vi "for testing.vi"() -> ()   [LabVIEW 2016] (continued)
            n234 = call "uc480_Error_Handling.vi"("Error Code"=w445, "Error String"=w454, "Error In"=w443) -> ("Error Out"=w447:errorcluster)  [unwired: 8 in]
          }
          frame True {
          }
        }
        n235 = call "uc480_SubVI_Example_MemoryAllocation.vi"(".NET (Reference)"=w406, "Error In"=w431) -> ("Error Out"=w408:errorcluster)  [unwired: 13 in, 4 out]
        n236 = call "uc480_SubVI_Example_GetPixelClock.vi"(".NET (Reference)"=w406, "Error In"=w408) -> ("Pixel Clock"=w409:i32, "Inc"=w411:i32, "Min"=w412:i32, "Max"=w413:i32, "error out"=w410:errorcluster)  [unwired: 9 in]
        n237 = property on="Pixelclock" class="Slide (strict)"(error in=w410, "Value"=w409, "Increment"=w411, "Minimum"=w412, "Maximum"=w413) -> (error out=w414:errorcluster)  [unwired: 1 in, 1 out]
        n238 = property on="Pixelclock" class="Slide (strict)"(error in=w414, "Scale.Increment"=w411, "Scale.Minimum"=w412, "Scale.Maximum"=w413) -> (error out=w415:errorcluster)  [unwired: 1 in, 1 out]
        n239 = call "uc480_SubVI_Example_GetFramerate.vi"(".NET (Reference)"=w406, "Error In"=w415) -> ("Framerate"=w418:dbl, "Inc"=w419:dbl, "Min"=w420:dbl, "Max"=w421:dbl, "error out"=w417:errorcluster)  [unwired: 9 in]
        n240 = property on="Framerate" class="Slide (strict)"(error in=w417, "Value"=w418, "Increment"=w419, "Minimum"=w420, "Maximum"=w421) -> (error out=w416:errorcluster)  [unwired: 1 in, 1 out]
        n241 = property on="Framerate" class="Slide (strict)"(error in=w416, "Scale.Increment"=w419, "Scale.Minimum"=w420, "Scale.Maximum"=w421) -> (error out=w422:errorcluster)  [unwired: 1 in, 1 out]
        n242 = call "uc480_SubVI_Example_GetExposure.vi"(".NET (Reference)"=w406, "Error In"=w422) -> ("Exposure"=w425:dbl, "Inc"=w426:dbl, "Min"=w427:dbl, "Max"=w428:dbl, "Error out"=w423:errorcluster)  [unwired: 9 in]
        n243 = property on="Exposure" class="Slide (strict)"(error in=w423, "Value"=w425, "Increment"=w426, "Minimum"=w427, "Maximum"=w428) -> (error out=w424:errorcluster)  [unwired: 1 in, 1 out]
        n244 = property on="Exposure" class="Slide (strict)"(error in=w424, "Scale.Increment"=w426, "Scale.Minimum"=w427, "Scale.Maximum"=w428) -> (error out=w407:errorcluster)  [unwired: 1 in, 1 out]
      }
      frame "Stop live" {
        # "Is acquisition running?"
        # "Stop Acquisition"
        n245 = property class="Camera"(reference=w472, error in=w473) -> (error out=w480:errorcluster, "Acquisition"=w479:refnum<k24>)  [unwired: 1 out]
        n246 = invoke class="Acquisition" method="HasStarted"(reference=w479, error in=w480) -> (reference out=w474:refnum<k24>, error out=w476:errorcluster, "bValue"=w478:bool)  [unwired: 2 in, 1 out]
        n247 = control-ref of="Load Parameter"() -> (w468:refnum<vi>)
        n248 = control-ref of="Start Live"() -> (w465:refnum<vi>)
        n249 = invoke class="Acquisition" method="ToString"(reference=w474, error in=w476) -> (reference out=w457:refnum<k24>, error out=w459:errorcluster, "ToString"=w475:string)  [unwired: 1 in]
        n250 = property class="Bool"(reference=w468, "Disabled"=u8 0 ("Deaktiviert")) -> (reference out=w463:refnum<vi>, error out=w462:errorcluster)  [unwired: 1 in]
        n251 = property class="Bool"(reference=w465, "Disabled"=u8 0 ("Deaktiviert")) -> (reference out=w461:refnum<vi>, error out=w460:errorcluster)  [unwired: 1 in]
        n252 = Close Reference(reference=w457, error in (no error)=w459) -> (error out=w458:errorcluster)
        n253 = Close Reference(reference=w463, error in (no error)=w462) -> ()  [unwired: 1 out]
        n254 = Close Reference(reference=w461, error in (no error)=w460) -> ()  [unwired: 1 out]
        n255 = call "uc480_Error_Handling.vi"("Error String"=w475, "Error In"=w458) -> ("Error Out"=w477:errorcluster)  [unwired: 9 in]
        n256 = case shown="True" w478 {
          tunnel: [w482 w501] -> w470
          tunnel: w477 -> [w482 w502]
          tunnel: w472 -> [w481 w494]
          tunnel: [w481 w494] -> w471
          frame False {
          }
          frame True {
            n257 = property class="Camera"(reference=w494, error in=w502) -> (error out=w498:errorcluster, "Acquisition"=w499:refnum<k24>)  [unwired: 1 out]
            n258 = invoke class="Acquisition" method="Stop"(reference=w499, error in=w498) -> (reference out=w496:refnum<k24>, error out=w497:errorcluster, "Stop"=w495:i32)  [unwired: 1 in]
            n259 = invoke class="Acquisition" method="ToString"(reference=w496, error in=w497) -> (reference out=w491:refnum<k24>, error out=w493:errorcluster, "ToString"=w500:string)  [unwired: 1 in]
            n260 = Close Reference(reference=w491, error in (no error)=w493) -> (error out=w492:errorcluster)
            n261 = call "uc480_Error_Handling.vi"("Error Code"=w495, "Error String"=w500, "Error In"=w492) -> ("Error Out"=w501:errorcluster)  [unwired: 8 in]
            n262 = Get Date/Time In Seconds() -> (seconds since 1Jan1904=w489:timestamp)
            n263 = Format Date/Time String(time format string (%c)="%m/%d/%y - %I:%M %p  ", seconds (now)=w489) -> (date/time string=w490:string)  [unwired: 1 in]
            n264 = Concatenate Strings(w490, "Camera stopped", "\r") -> (w485:string)
            n265 = invoke on="Log" class="Str" method="Append String"("string"=w485) -> (error out=w483:errorcluster)  [unwired: 3 in, 3 out]
            n266 = property on="Log" class="Str"(error in=w483, "Text.Scroll Position"=u32 500000) -> ()  [unwired: 1 in, 2 out]
          }
        }
      }
      frame "Exit camera" {
        # "Close .Net Reference"
        # "Is acquisition running?"
        # "Stop Acquisition"
        # "Close Camera"
        n267 = property class="Camera"(reference=w530, error in=w531) -> (error out=w538:errorcluster, "Acquisition"=w537:refnum<k24>)  [unwired: 1 out]
        n268 = invoke class="Acquisition" method="HasStarted"(reference=w537, error in=w538) -> (reference out=w532:refnum<k24>, error out=w534:errorcluster, "bValue"=w536:bool)  [unwired: 2 in, 1 out]
        n269 = control-ref of="Load Parameter"() -> (w521:refnum<vi>)
        n270 = control-ref of="Init Camera"() -> (w523:refnum<vi>)
        n271 = control-ref of="Start Live"() -> (w522:refnum<vi>)
        n272 = control-ref of="Stop Live"() -> (w520:refnum<vi>)
        n273 = invoke class="Acquisition" method="ToString"(reference=w532, error in=w534) -> (reference out=w517:refnum<k24>, error out=w519:errorcluster, "ToString"=w533:string)  [unwired: 1 in]
        n274 = property class="Bool"(reference=w522, "Disabled"=u8 0 ("Deaktiviert")) -> (reference out=w506:refnum<vi>, error out=w505:errorcluster)  [unwired: 1 in]
        n275 = property class="Bool"(reference=w523, "Disabled"=u8 0 ("Deaktiviert")) -> (reference out=w504:refnum<vi>, error out=w503:errorcluster)  [unwired: 1 in]
        n276 = property class="Bool"(reference=w521, "Disabled"=u8 0 ("Deaktiviert")) -> (reference out=w508:refnum<vi>, error out=w507:errorcluster)  [unwired: 1 in]
        n277 = property class="Bool"(reference=w520, "Disabled"=u8 0 ("Deaktiviert")) -> (reference out=w510:refnum<vi>, error out=w509:errorcluster)  [unwired: 1 in]
        n278 = Close Reference ("Close Referenz")(reference=w517, error in (no error)=w519) -> (error out=w518:errorcluster)
        n279 = Close Reference(reference=w506, error in (no error)=w505) -> ()  [unwired: 1 out]
        n280 = Close Reference(reference=w504, error in (no error)=w503) -> ()  [unwired: 1 out]
        n281 = Close Reference(reference=w510, error in (no error)=w509) -> ()  [unwired: 1 out]
        n282 = Close Reference(reference=w508, error in (no error)=w507) -> ()  [unwired: 1 out]
        n283 = call "uc480_Error_Handling.vi"("Error String"=w533, "Error In"=w518) -> ("Error Out"=w535:errorcluster)  [unwired: 9 in]
        n284 = case shown="True" w536 {
          tunnel: [w547 w558] -> w528
          tunnel: w535 -> [w547 w559]
          tunnel: w530 -> [w546 w551]
          tunnel: [w546 w551] -> w529
          frame False {
          }
          frame True {
            n285 = property class="Camera"(reference=w551, error in=w559) -> (error out=w555:errorcluster, "Acquisition"=w556:refnum<k24>)  [unwired: 1 out]
            n286 = invoke class="Acquisition" method="Stop"(reference=w556, error in=w555) -> (reference out=w553:refnum<k24>, error out=w554:errorcluster, "Stop"=w552:i32)  [unwired: 1 in]
            n287 = invoke class="Acquisition" method="ToString"(reference=w553, error in=w554) -> (reference out=w548:refnum<k24>, error out=w550:errorcluster, "ToString"=w557:string)  [unwired: 1 in]
            n288 = Close Reference ("Close Referenz")(reference=w548, error in (no error)=w550) -> (error out=w549:errorcluster)
            n289 = call "uc480_Error_Handling.vi"("Error Code"=w552, "Error String"=w557, "Error In"=w549) -> ("Error Out"=w558:errorcluster)  [unwired: 8 in]
          }
        }
        n290 = invoke class="Camera" method="Exit"(reference=w529, error in=w528) -> (reference out=w539:refnum<k24>, error out=w542:errorcluster, "Exit"=w541:i32)  [unwired: 1 in]
        n291 = invoke class="Camera" method="ToString"(reference=w539, error in=w542) -> (error out=w543:errorcluster, "ToString"=w544:string)  [unwired: 1 in, 1 out]
        n292 = call "uc480_Error_Handling.vi"("Error Code"=w541, "Error String"=w544, "Error In"=w543) -> ("Error Out"=w516:errorcluster)  [unwired: 8 in]
        n293 = property class="PictureBox"(reference=w512, error in=w516, "Width"=853, "Height"=682) -> (reference out=w511:refnum<k24>, error out=w515:errorcluster)
        n294 = Close Reference ("Close Referenz")(reference=w539, error in (no error)=w515) -> (error out=w540:errorcluster)
      }
      frame Default {
        # "SubVI Example for Timing"
        # "Has acquisition started?"
        n295 = call "uc480_SubVI_Example_Timing.vi"(".NET (Reference)"=w572, "Pixelclock"="Pixelclock", "Exposure time"="Exposure", "Framerate"="Framerate", "Error In"=w582) -> ("Pixelclock"=w575:i32, "Exposure time"=w574:dbl, "Framerate"=w573:dbl, "Error Out"=w579:errorcluster)  [unwired: 7 in]
        n296 = property on="Framerate" class="Schieber (strikt)"(error in=w579, "Scale.RngStart"=w573) -> (error out=w578:errorcluster)  [unwired: 1 in, 1 out]
        n297 = property on="Exposure" class="Schieber (strikt)"(error in=w578, "Scale.RngStart"=w574) -> (error out=w577:errorcluster)  [unwired: 1 in, 1 out]
        n298 = property on="Pixelclock" class="Schieber (strikt)"(error in=w577, "Scale.RngStart"=w575) -> (error out=w576:errorcluster)  [unwired: 1 in, 1 out]
        n299 = property class="Camera"(reference=w572, error in=w576) -> (reference out=w565:refnum<k24>, error out=w588:errorcluster, "Acquisition"=w587:refnum<k24>)
        n300 = invoke class="Acquisition" method="HasStarted"(reference=w587, error in=w588) -> (reference out=w562:refnum<k24>, error out=w584:errorcluster, "HasStarted"=w583:i32, "bValue"=w561:bool)  [unwired: 2 in]
        n301 = invoke class="Acquisition" method="ToString"(reference=w562, error in=w584) -> (reference out=w566:refnum<k24>, error out=w586:errorcluster, "ToString"=w585:string)  [unwired: 1 in]
        n302 = call "uc480_Error_Handling.vi"("Error Code"=w583, "Error String"=w585, "Error In"=w586) -> ("Error Out"=w568:errorcluster)  [unwired: 8 in]
        n303 = Close Reference(reference=w566, error in (no error)=w568) -> (error out=w567:errorcluster)
        n304 = case "Show Image" shown="True" w561 {
          tunnel: [w592 w604] -> w580
          tunnel: w567 -> [w592 w632]
          tunnel: w565 -> [w591 w596]
          tunnel: [w591 w600] -> w581
          tunnel: w564 -> [w590 w621]
          tunnel: [w590 w598] -> w563
          tunnel: w560 -> [_ w628]
          frame False {
            (unwired) ""
          }
          frame True {
            n305 = local read "Height"() -> (w625:i32)
            n306 = local read "Width"() -> (w626:i32)
            n307 = Quotient & Remainder(x=w626, y="Zoom") -> (floor(x/y)=w623:dbl)  [unwired: 1 out]
            n308 = Quotient & Remainder(x=w625, y="Zoom") -> (floor(x/y)=w622:dbl)  [unwired: 1 out]
            n309 = To Long Integer(number=w623) -> (32bit integer=w595:i32)
            n310 = To Long Integer(number=w622) -> (32bit integer=w594:i32)
            n311 = property class="PictureBox"(reference=w621, error in=w632, "Width"=w595, "Height"=w594) -> (reference out=w598:refnum<k24>, error out=w627:errorcluster)
            n312 = property class="Camera"(reference=w596, error in=w627) -> (reference out=w597:refnum<k24>, error out=w634:errorcluster, "Memory"=w635:refnum<k24>)
            n313 = invoke class="Memory" method="GetActive"(reference=w635, error in=w634) -> (reference out=w629:refnum<k24>, error out=w630:errorcluster, "s32MemId"=w601:i32)  [unwired: 2 in, 1 out]
            n314 = property class="Camera"(reference=w597, error in=w630) -> (reference out=w609:refnum<k24>, error out=w633:errorcluster, "Display"=w618:refnum<k24>)
            n315 = invoke class="Display" method="Render"(reference=w618, error in=w633, "memID"=w601, "windowHandle"=w628) -> (reference out=w619:refnum<k24>, error out=w620:errorcluster)  [unwired: 1 in, 3 out]
            n316 = property class="Camera"(reference=w609, error in=w620) -> (reference out=w600:refnum<k24>, error out=w616:errorcluster, "Gain"=w614:refnum<k24>)
            n317 = property class="Gain"(reference=w614, error in=w616) -> (reference out=w615:refnum<k24>, error out=w611:errorcluster, "Hardware"=w610:refnum<k24>)
            n318 = property class="GainHardware"(reference=w610, error in=w611) -> (reference out=w607:refnum<k24>, error out=w612:errorcluster, "Boost"=w613:refnum<k24>)
            n319 = property class="GainBoost"(reference=w613, error in=w612, "Enabled"="Gain Boost") -> (reference out=w608:refnum<k24>, error out=w599:errorcluster)
            n320 = case "Snapshot control" shown="True" "Snapshot" {
              tunnel: w596 -> [_ w656]
              tunnel: w599 -> [w636 w660]
              tunnel: [w636 w647] -> w593
              tunnel: w595 -> [_ w650]
              tunnel: w594 -> [_ w649]
              frame False {
              }
              frame True {
                n321 = property class="Camera"(reference=w656, error in=w660) -> (error out=w680:errorcluster, "Memory"=w679:refnum<k24>)  [unwired: 1 out]
                n322 = local read "Zoom"() -> (w655:dbl)
                n323 = invoke class="Memory" method="GetList"(reference=w679, error in=w680) -> (reference out=w685:refnum<k24>, error out=w684:errorcluster, "GetList"=w686:i32, "idList"=w673:i32[])  [unwired: 2 in]
                n324 = Bundle(cluster=T7 {"Width"=0, "Height"=0} ("Draw Area Size"), "Width"=w650, "Height"=w649) -> (w651:T7)
                n325 = Divide(x=1.0, y=w655) -> (x/y=w653:dbl)
                n326 = property on="Output" class="Pict"("ZoomFactor"=w653, "Draw Area Size"=w651) -> ()  [unwired: 2 in, 2 out]
                n327 = invoke class="Memory" method="ToString"(reference=w685, error in=w684) -> (reference out=w658:refnum<k24>, error out=w668:errorcluster, "ToString"=w683:string)  [unwired: 1 in]
                n328 = Index Array(array=w673, index=0 ("Active \nAcquisition Buffer")) -> (element=w670:i32)
                n329 = Index Array(array=w673, index=u32 0 ("Active \nOutput Buffer")) -> (element=w669:i32)
                n330 = Close Reference(reference=w658, error in (no error)=w668) -> (error out=w667:errorcluster)
                n331 = call "uc480_Error_Handling.vi"("Error Code"=w686, "Error String"=w683, "Error In"=w667) -> ("Error Out"=w676:errorcluster)  [unwired: 8 in]
                n332 = Get Date/Time In Seconds() -> (seconds since 1Jan1904=w640:timestamp)
                n333 = property class="Camera"(reference=w656, error in=w676) -> (error out=w675:errorcluster, "Memory"=w674:refnum<k24>)  [unwired: 1 out]
                n334 = Format Date/Time String(time format string (%c)="%m/%d/%y -%I:%M %p  ", seconds (now)=w640) -> (date/time string=w639:string)  [unwired: 1 in]
                n335 = invoke class="Memory" method="SetActive"(reference=w674, error in=w675, "s32MemId"=w670) -> (reference out=w659:refnum<k24>, error out=w666:errorcluster)  [unwired: 1 in, 2 out]
                n336 = Concatenate Strings(w639, "Snapshot taken", "\r") -> (w644:string)
                n337 = Close Reference(reference=w659, error in (no error)=w666) -> (error out=w665:errorcluster)
                n338 = invoke on="Log" class="Str" method="Append String"("string"=w644) -> (error out=w637:errorcluster)  [unwired: 3 in, 3 out]
                n339 = property class="Camera"(reference=w656, error in=w665) -> (error out=w682:errorcluster, "Memory"=w671:refnum<k24>)  [unwired: 1 out]
                n340 = invoke class="Memory" method="CopyToArray"(reference=w671, error in=w682, "s32MemId"=w669) -> (reference out=w661:refnum<k24>, error out=w662:errorcluster, "u8Image"=w681:u8[])  [unwired: 2 in, 2 out]
                n341 = property on="Log" class="Str"(error in=w637, "Text.Scroll Position"=u32 500000) -> ()  [unwired: 1 in, 2 out]
                n342 = invoke class="Memory" method="ToString"(reference=w661, error in=w662) -> (reference out=w657:refnum<k24>, error out=w664:errorcluster, "ToString"=w687:string)  [unwired: 1 in]
                n343 = Close Reference(reference=w657, error in (no error)=w664) -> (error out=w663:errorcluster)
                n344 = call "uc480_Error_Handling.vi"("Error String"=w687, "Error In"=w663) -> ("Error Out"=w678:errorcluster)  [unwired: 9 in]
                n345 = call "uc480_ArrayToImage.vi"("Error In"=w678, "InArray"=w681, ".NET (Reference)"=w656) -> ("Error Out"=w646:errorcluster, "Image"=w648:picture)  [unwired: 7 in]
                "Output" <- w648
                n346 = call "Picture to IMAQ.vi"("Error In"=w646, "picture"=w648) -> ("Error Out"=w647:errorcluster, "Image"=→"Source":T1)  [unwired: 8 in]
              }
            }
            n347 = Close Reference(reference=w607, error in (no error)=w593) -> (error out=w606:errorcluster)
            n348 = Close Reference(reference=w608, error in (no error)=w606) -> (error out=w603:errorcluster)
            n349 = Close Reference(reference=w615, error in (no error)=w603) -> (error out=w617:errorcluster)
            n350 = Close Reference(reference=w619, error in (no error)=w617) -> (error out=w631:errorcluster)
            n351 = Close Reference(reference=w629, error in (no error)=w631) -> (error out=w604:errorcluster)
          }
        }
      }
      frame "Init camera" {
        # "SubVI Example for \nGetDefault Timing"
        # "SubVI Example for \nMemory allocation"
        # "SubVI Example for \nTiming"
        # "SubVI Example for \nCamera Init"
        # "Pixelformat"
        n352 = control-ref of="Load Parameter"() -> (w711:refnum<vi>)
        n353 = call "uc480_SubVI_Example_CameraInit.vi"("Error In"=w751, "Camera ID"="Camera ID", "Init Camera Flag"=TRUE, ".NET (Reference)"=w752) -> ("Error Out"=w757:errorcluster, ".NET (Reference)"=w710:refnum<k24>)  [unwired: 6 in]
        n354 = control-ref of="Init Camera"() -> (w715:refnum<vi>)
        n355 = control-ref of="Start Live"() -> (w713:refnum<vi>)
        n356 = property on="Property Node" class="Camera"(reference=w710, error in=w757) -> (error out=w758:errorcluster, "PixelFormat"=w759:refnum<k24>)  [unwired: 1 out]
        n357 = property class="Bool"(reference=w713, "Disabled"=u8 0 ("Deaktiviert")) -> (reference out=w702:refnum<vi>, error out=w701:errorcluster)  [unwired: 1 in]
        n358 = property class="Bool"(reference=w715, "Disabled"=u8 2 ("Deaktiviert")) -> (reference out=w704:refnum<vi>, error out=w703:errorcluster)  [unwired: 1 in]
        n359 = property class="Bool"(reference=w711, "Disabled"=u8 0 ("Deaktiviert")) -> (reference out=w700:refnum<vi>, error out=w699:errorcluster)  [unwired: 1 in]
        n360 = Close Reference(reference=w702, error in (no error)=w701) -> ()  [unwired: 1 out]
        n361 = Close Reference(reference=w704, error in (no error)=w703) -> ()  [unwired: 1 out]
        n362 = Close Reference(reference=w700, error in (no error)=w699) -> ()  [unwired: 1 out]
        n363 = invoke class="PixelFormat" method="Set"(reference=w759, error in=w758, "mode"="Mode") -> (reference out=w755:refnum<k24>, error out=w748:errorcluster, "Set"=w754:i32)  [unwired: 1 in, 1 out]
        n364 = Get Date/Time In Seconds() -> (seconds since 1Jan1904=w691:timestamp)
        n365 = Format Date/Time String(time format string (%c)="%m/%d/%y - %I:%M %p  ", seconds (now)=w691) -> (date/time string=w690:string)  [unwired: 1 in]
        n366 = invoke class="PixelFormat" method="ToString"(reference=w755, error in=w748) -> (reference out=w696:refnum<k24>, error out=w698:errorcluster, "ToString"=w756:string)  [unwired: 1 in]
        n367 = Concatenate Strings(w690, "Camera Initialized", "\r") -> (w695:string)
        n368 = Close Reference(reference=w696, error in (no error)=w698) -> (error out=w697:errorcluster)
        n369 = call "uc480_Error_Handling.vi"("Error Code"=w754, "Error String"=w756, "Error In"=w697) -> ("Error Out"=w722:errorcluster)  [unwired: 8 in]
        n370 = invoke on="Log" class="Str" method="Append String"("string"=w695) -> (error out=w688:errorcluster)  [unwired: 3 in, 3 out]
        n371 = property on="Log" class="Str"(error in=w688, "Text.Scroll Position"=u32 500000) -> ()  [unwired: 1 in, 2 out]
        n372 = call "uc480_SubVI_Example_GetDefault_Timing.vi"(".NET (Reference)"=w710, "Error In"=w722) -> ("Pixelclock"=w721:i32, "Exposure time"=w720:dbl, "Framerate"=w719:dbl, "Error Out"=w718:errorcluster)  [unwired: 10 in]
        n373 = call "uc480_SubVI_Example_GetPixelClock.vi"(".NET (Reference)"=w710, "Error In"=w718) -> ("Pixel Clock"=w723:i32, "Inc"=w725:i32, "Min"=w726:i32, "Max"=w727:i32, "error out"=w724:errorcluster)  [unwired: 9 in]
        n374 = property on="Pixelclock" class="Slide (strict)"(error in=w724, "Value"=w723, "Increment"=w725, "Minimum"=w726, "Maximum"=w727) -> (error out=w728:errorcluster)  [unwired: 1 in, 1 out]
        n375 = property on="Pixelclock" class="Slide (strict)"(error in=w728, "Scale.Increment"=w725, "Scale.Minimum"=w726, "Scale.Maximum"=w727) -> (error out=w729:errorcluster)  [unwired: 1 in, 1 out]
        n376 = call "uc480_SubVI_Example_GetFramerate.vi"(".NET (Reference)"=w710, "Error In"=w729) -> ("Framerate"=w732:dbl, "Inc"=w733:dbl, "Min"=w734:dbl, "Max"=w735:dbl, "error out"=w731:errorcluster)  [unwired: 9 in]
        n377 = property on="Framerate" class="Slide (strict)"(error in=w731, "Value"=w732, "Increment"=w733, "Minimum"=w734, "Maximum"=w735) -> (error out=w730:errorcluster)  [unwired: 1 in, 1 out]
        n378 = property on="Framerate" class="Slide (strict)"(error in=w730, "Scale.Increment"=w733, "Scale.Minimum"=w734, "Scale.Maximum"=w735) -> (error out=w736:errorcluster)  [unwired: 1 in, 1 out]
        n379 = call "uc480_SubVI_Example_GetExposure.vi"(".NET (Reference)"=w710, "Error In"=w736) -> ("Exposure"=w739:dbl, "Inc"=w740:dbl, "Min"=w741:dbl, "Max"=w742:dbl, "Error out"=w737:errorcluster)  [unwired: 9 in]
        n380 = property on="Exposure" class="Slide (strict)"(error in=w737, "Value"=w739, "Increment"=w740, "Minimum"=w741, "Maximum"=w742) -> (error out=w738:errorcluster)  [unwired: 1 in, 1 out]
        n381 = property on="Exposure" class="Slide (strict)"(error in=w738, "Scale.Increment"=w740, "Scale.Minimum"=w741, "Scale.Maximum"=w742) -> (error out=w717:errorcluster)  [unwired: 1 in, 1 out]
        n382 = call "uc480_SubVI_Example_Timing.vi"(".NET (Reference)"=w710, "Pixelclock"=w721, "Exposure time"=w720, "Framerate"=w719, "Error In"=w717) -> ("Error Out"=w709:errorcluster)  [unwired: 7 in, 3 out]
        n383 = call "uc480_SubVI_Example_Is_XS.vi"("Error In"=w709, ".NET (Reference)"=w710) -> ("Error Out"=w706:errorcluster, "IsXS"=w708:bool)  [unwired: 7 in, 1 out]
        n384 = case shown="False" w708 {
          tunnel: w706 -> [w773 w786]
          tunnel: [w773 w786] -> w707
          frame False {
            n385 = control-ref of="Pixelclock"() -> (w769:refnum<vi>)
            n386 = control-ref of="Framerate"() -> (w768:refnum<vi>)
            n387 = control-ref of="Exposure"() -> (w767:refnum<vi>)
            n388 = property class="Slide (strict)"(reference=w769, "DisabledEnum"=T8."Enabled" ("Disabled")) -> (reference out=w766:refnum<vi>, error out=w765:errorcluster)  [unwired: 1 in]
            n389 = property class="Slide (strict)"(reference=w768, "DisabledEnum"=T8."Enabled" ("Disabled")) -> (reference out=w764:refnum<vi>, error out=w763:errorcluster)  [unwired: 1 in]
            n390 = property class="Slide (strict)"(reference=w767, "DisabledEnum"=T8."Enabled" ("Disabled")) -> (reference out=w762:refnum<vi>, error out=w761:errorcluster)  [unwired: 1 in]
            n391 = Close Reference(reference=w766, error in (no error)=w765) -> ()  [unwired: 1 out]
            n392 = Close Reference(reference=w764, error in (no error)=w763) -> ()  [unwired: 1 out]
            n393 = Close Reference(reference=w762, error in (no error)=w761) -> ()  [unwired: 1 out]
          }
          frame True {
            n394 = control-ref of="Pixelclock"() -> (w785:refnum<vi>)
            n395 = control-ref of="Framerate"() -> (w782:refnum<vi>)
            n396 = control-ref of="Exposure"() -> (w780:refnum<vi>)
            n397 = property class="Slide (strict)"(reference=w785, "DisabledEnum"=T8."Disabled and Grayed Out" ("Disabled")) -> (reference out=w778:refnum<vi>, error out=w779:errorcluster)  [unwired: 1 in]
            n398 = property class="Slide (strict)"(reference=w782, "DisabledEnum"=T8."Disabled and Grayed Out" ("Disabled")) -> (reference out=w777:refnum<vi>, error out=w776:errorcluster)  [unwired: 1 in]
            n399 = property class="Slide (strict)"(reference=w780, "DisabledEnum"=T8."Disabled and Grayed Out" ("Disabled")) -> (reference out=w775:refnum<vi>, error out=w774:errorcluster)  [unwired: 1 in]
            n400 = Close Reference(reference=w778, error in (no error)=w779) -> ()  [unwired: 1 out]
            n401 = Close Reference(reference=w777, error in (no error)=w776) -> ()  [unwired: 1 out]
            n402 = Close Reference(reference=w775, error in (no error)=w774) -> ()  [unwired: 1 out]
          }
        }
        n403 = call "uc480_SubVI_Example_MemoryAllocation.vi"(".NET (Reference)"=w710, "Error In"=w707) -> ("Bits/Pixel 2"=→"Bits/Pixel":i32, "Width"=→"Width":i32, "Serial Number"=→"Serial Number":string, "Height"=→"Height":i32, "Error Out"=w747:errorcluster)  [unwired: 13 in]
      }
      frame "Start live" {
        # "Has acquisition started?"
        # "Start Acquisition"
        n404 = property class="Camera"(reference=w811, error in=w812) -> (error out=w821:errorcluster, "Acquisition"=w820:refnum<k24>)  [unwired: 1 out]
        n405 = invoke class="Acquisition" method="HasStarted"(reference=w820, error in=w821) -> (reference out=w816:refnum<k24>, error out=w815:errorcluster, "HasStarted"=w814:i32, "bValue"=w819:bool)  [unwired: 2 in]
        n406 = control-ref of="Load Parameter"() -> (w804:refnum<vi>)
        n407 = control-ref of="Stop Live"() -> (w802:refnum<vi>)
        n408 = control-ref of="Start Live"() -> (w807:refnum<vi>)
        n409 = property class="Bool"(reference=w807, "Disabled"=u8 2 ("Deaktiviert")) -> (reference out=w796:refnum<vi>, error out=w795:errorcluster)  [unwired: 1 in]
        n410 = property class="Bool"(reference=w804, "Disabled"=u8 2 ("Deaktiviert")) -> (reference out=w798:refnum<vi>, error out=w797:errorcluster)  [unwired: 1 in]
        n411 = invoke class="Acquisition" method="ToString"(reference=w816, error in=w815) -> (error out=w818:errorcluster, "ToString"=w817:string)  [unwired: 1 in, 1 out]
        n412 = property class="Bool"(reference=w802, "Disabled"=u8 0 ("Deaktiviert")) -> (reference out=w800:refnum<vi>, error out=w799:errorcluster)  [unwired: 1 in]
        n413 = call "uc480_Error_Handling.vi"("Error Code"=w814, "Error String"=w817, "Error In"=w818) -> ("Error Out"=w813:errorcluster)  [unwired: 8 in]
        n414 = Close Reference(reference=w800, error in (no error)=w799) -> ()  [unwired: 1 out]
        n415 = Close Reference(reference=w796, error in (no error)=w795) -> ()  [unwired: 1 out]
        n416 = Close Reference(reference=w798, error in (no error)=w797) -> ()  [unwired: 1 out]
        n417 = Get Date/Time In Seconds() -> (seconds since 1Jan1904=w790:timestamp)
        n418 = Format Date/Time String(time format string (%c)="%m/%d/%y - %I:%M %p  ", seconds (now)=w790) -> (date/time string=w789:string)  [unwired: 1 in]
        n419 = Concatenate Strings(w789, "Camera started", "\r") -> (w794:string)
        n420 = invoke on="Log" class="Str" method="Append String"("string"=w794) -> (error out=w787:errorcluster)  [unwired: 3 in, 3 out]
        n421 = property on="Log" class="Str"(error in=w787, "Text.Scroll Position"=u32 500000) -> ()  [unwired: 1 in, 2 out]
        n422 = case shown="False" w819 {
          tunnel: [w824 w834] -> w808
          tunnel: w813 -> [w830 w834]
          tunnel: w811 -> [w829 w833]
          tunnel: [w829 w833] -> w810
          frame False {
            w822 = 1 items=["IS_DONT_WAIT", "IS_WAIT"] ("Wait")
            n423 = property class="Camera"(reference=w829, error in=w830) -> (error out=w831:errorcluster, "Acquisition"=w832:refnum<k24>)  [unwired: 1 out]
            n424 = invoke class="Acquisition" method="Capture"(reference=w832, error in=w831, "param"=w822) -> (reference out=w825:refnum<k24>, error out=w826:errorcluster, "Capture"=w823:i32)  [unwired: 1 in, 1 out]
            n425 = invoke class="Acquisition" method="ToString"(reference=w825, error in=w826) -> (error out=w828:errorcluster, "ToString"=w827:string)  [unwired: 1 in, 1 out]
            n426 = call "uc480_Error_Handling.vi"("Error Code"=w823, "Error String"=w827, "Error In"=w828) -> ("Error Out"=w824:errorcluster)  [unwired: 8 in]
          }
          frame True {
          }
        }
      }
    }
    n427 = call "uc480_SubVI_Example_SyncEventLoop.vi"("Error In"=w348, "use sync"=w350, ".NET (Reference)"=w349) -> ("Error Out"=w346:errorcluster, "Synchronize (ms)"=w347:dbl)  [unwired: 7 in]
    "Error Out" <- w346
    n428 = Wait Until Next ms Multiple(millisecond multiple=w347) -> ()  [unwired: 1 out]
  }
  n429 = while "Laser control & Stages Control" {
    stop <- w845 stop-if-true
    n430 = local read "XPS_Address"() -> (w837:string)
    n431 = local read "Axis 2"() -> (w835:string)
    n432 = local read "Axis 1"() -> (w836:string)
    n433 = event shown="[13] \"Transparency\": Value Change" {
      selector: _ -> [_ _ _ _ _ _ _ _ _ _ _ _ _ _ _]
      dyn-events: _ -> [_ _ _ _ _ _ _ _ _ _ _ _ _ _ _]
      timeout: _ -> [_ _ _ _ _ _ _ _ _ _ _ _ _ _ _]
      tunnel: [_ _ _ _ _ w917 _ _ _ _ _ _ _ _ _] -> w845
      tunnel: [w849 w856 w875 w898 w905 _ _ _ w955 w980 _ "" ("StringOut") w1137 _ w1261] -> w838
      tunnel: w837 -> [_ _ _ _ _ _ _ _ _ w983 _ w1056 w1136 _ w1248]
      tunnel: w836 -> [_ _ _ _ _ _ _ _ _ w982 _ w1055 w1135 _ w1247]
      tunnel: w835 -> [_ _ _ _ _ _ _ _ _ w981 _ w1054 w1134 _ w1246]
      event "Flash lamp - Q Switch delay (%)": Value Change {
        n434 = event-data() -> ()  [unwired: 1 in, 6 out]
        n435 = local read "Flash lamp - Q Switch delay (%)"() -> (w853:i16)
        n436 = call "IR_Laser_Control.vi"("Action"=T9."Adjust Energy", "Energy (0 - 100)"=w853) -> ()  [unwired: 13 in, 1 out]
        n437 = Number To Decimal String(number=w853, width (-)=i16 3) -> (decimal integer string=w851:string)
        n438 = Concatenate Strings("Energy set to: " ("string"), w851) -> (w849:string)
      }
      event "LAMP": Value Change {
        n439 = event-data() -> ()  [unwired: 1 in, 6 out]
        n440 = case shown="True" "LAMP" {
          tunnel: ["Lamp has been switched off" w861] -> w856
          frame False {
            w858 = FALSE ("Visible")
            n441 = property on="LASER" class="Bool (strict)"("Visible"=w858) -> ()  [unwired: 2 in, 2 out]
            n442 = property on="Capture" class="Bool"("Visible"=w858) -> ()  [unwired: 2 in, 2 out]
            n443 = call "IR_Laser_Control.vi"("Action"=T9."Lamp OFF") -> ()  [unwired: 14 in, 1 out]
            n444 = property on="LAMP" class="Bool (strict)"("BoolText.Text"="LAMP OFF" ("Boolean Text.Text")) -> ()  [unwired: 2 in, 2 out]
          }
          frame True {
            n445 = flat-sequence {
              tunnel: ["Lamp has been switched on"] -> w861
              frame #0 {
                n446 = while {
                  i -> [w866]
                  stop <- w869 stop-if-true
                  n447 = Wait Until Next ms Multiple(millisecond multiple=u32 1000) -> ()  [unwired: 1 out]
                  n448 = Equal?(x=10, y=w866) -> (x = y?=w869:bool)
                  n449 = Subtract(x=10, y=w866) -> (x-y=w864:i32)
                  n450 = Number To Decimal String(number=w864) -> (decimal integer string=w865:string)  [unwired: 1 in]
                  n451 = property on="LAMP" class="Bool (strict)"("BoolText.Text"=w865) -> ()  [unwired: 2 in, 2 out]
                }
                n452 = Wait (ms)(milliseconds to wait=u32 10000) -> ()  [unwired: 1 out]
                n453 = call "IR_Laser_Control.vi"("Action"=T9."Lamp ON") -> ()  [unwired: 14 in, 1 out]
              }
              frame #1 {
                w872 = TRUE ("Visible")
                n454 = property on="LASER" class="Bool (strict)"("Visible"=w872) -> ()  [unwired: 2 in, 2 out]
                n455 = property on="Capture" class="Bool"("Visible"=w872) -> ()  [unwired: 2 in, 2 out]
                n456 = property on="LAMP" class="Bool (strict)"("BoolText.Text"="LAMP ON" ("Boolean Text.Text")) -> ()  [unwired: 2 in, 2 out]
              }
            }
          }
        }
      }
      event "LASER": Value Change {
        n457 = event-data() -> ()  [unwired: 1 in, 6 out]
        n458 = case shown="True" "LASER" {
          tunnel: [w880 w886] -> w876
          tunnel: ["Q-Switch has switched off" w885] -> w875
          frame False {
            w880 = FALSE ("Boolean")
            n459 = property on="Capture" class="Bool"("Visible"=TRUE) -> ()  [unwired: 2 in, 2 out]
            n460 = local read "Alignment \ndiode"() -> (w877:bool)
            n461 = case shown="False" w877 {
              frame False {
                n462 = call "IR_Alignment_Diode.vi"("AD Action"=enum16{"AD Off", "AD On"}."AD Off") -> ()  [unwired: 14 in, 1 out]
              }
              frame True {
                n463 = call "IR_Alignment_Diode.vi"("AD Action"=enum16{"AD Off", "AD On"}."AD On") -> ()  [unwired: 14 in, 1 out]
              }
            }
            n464 = call "IR_Laser_Control.vi"("Action"=T9."Q-switch OFF") -> ()  [unwired: 14 in, 1 out]
            n465 = property on="LASER" class="Bool (strict)"("BoolText.Text"="LASER OFF" ("Boolean Text.Text"), "Value"=w880) -> ()  [unwired: 2 in, 2 out]
            n466 = property on="Laser Operation" class="Bool (strict)"("Blinking"=w880) -> ()  [unwired: 2 in, 2 out]
          }
          frame True {
            n467 = property on="LAMP" class="Bool (strict)"() -> ("BoolText.Text"=w889:string)  [unwired: 2 in, 2 out]
            n468 = Equal?(x=w889, y="LAMP ON") -> (x = y?=w887:bool)
            n469 = case shown="True" w887 {
              tunnel: [FALSE ("Boolean") w895] -> w886
              tunnel: ["Q-Switch has switched off" "Q-Switch has switched on"] -> w885
              frame False {
              }
              frame True {
                w895 = TRUE ("Boolean")
                n470 = property on="Capture" class="Bool"("Visible"=FALSE) -> ()  [unwired: 2 in, 2 out]
                n471 = call "IR_Alignment_Diode.vi"("AD Action"=enum16{"AD Off", "AD On"}."AD Off") -> ()  [unwired: 14 in, 1 out]
                n472 = property on="LASER" class="Bool (strict)"("BoolText.Text"="LASER ON" ("Boolean Text.Text")) -> ()  [unwired: 2 in, 2 out]
                n473 = property on="Laser Operation" class="Bool (strict)"("Blinking"=w895) -> ()  [unwired: 2 in, 2 out]
                n474 = call "IR_Laser_Control.vi"("Action"=T9."Q-switch ON") -> ()  [unwired: 14 in, 1 out]
              }
            }
          }
        }
        "Laser Operation" <- w876
      }
      event "Repetition \nRate": Value Change {
        n475 = event-data() -> ()  [unwired: 1 in, 6 out]
        n476 = local read "Repetition \nRate"() -> (w899:enum16{"1", "2", "5", "10", "20"})
        n477 = call "IR_Laser_Control.vi"("Action"=T9."Change Rep. Rate", "Rep. Rate Divider"=w899) -> ()  [unwired: 13 in, 1 out]
        n478 = Number To Decimal String(number=w899, width (-)=i16 3) -> (decimal integer string=w901:string)
        n479 = Concatenate Strings("Repetition rate set to: " ("string"), w901) -> (w898:string)
      }
      event "Tune": Value Change {
        n480 = event-data() -> ()  [unwired: 1 in, 6 out]
        n481 = case shown="True" "Tune" {
          tunnel: [_ w906] -> w905
          frame False {
          }
          frame True {
            n482 = property on="LASER" class="Bool (strict)"() -> ("BoolText.Text"=w913:string)  [unwired: 2 in, 2 out]
            n483 = Equal?(x=w913, y="LASER ON") -> (x = y?=w911:bool)
            n484 = case shown="False" w911 {
              tunnel: [w914 w915] -> w907
              frame False {
                n485 = local read "Wavelength"() -> (w914:dbl)
                n486 = call "IR_Wavelength_Tuning.vi"("Wavelength (nm)"=w914) -> ()  [unwired: 14 in, 1 out]
              }
              frame True {
                n487 = local read "Wavelength"() -> (w915:dbl)
              }
            }
            n488 = Number To Decimal String(number=w907, width (-)=i16 3) -> (decimal integer string=w909:string)
            n489 = Concatenate Strings("Wavelength set to: " ("string"), w909) -> (w906:string)
          }
        }
      }
      event "EXIT": Value Change {
        n490 = event-data() -> ()  [unwired: 1 in, 6 out]
        n491 = flat-sequence {
          tunnel: [w920] -> w916
          tunnel: w916 -> [w921]
          tunnel: ["EXIT"] -> w917
          frame #0 {
          }
          frame #1 {
          }
          frame #2 {
            n492 = local write "Camera Status"("Exit camera") -> ()
          }
          frame #3 {
            n493 = Wait (ms)(milliseconds to wait=u32 1000) -> ()  [unwired: 1 out]
          }
          frame #4 {
            w920 = TRUE ("Exit Camera")
            n494 = local write "EXIT 3"(w920) -> ()
          }
          frame #5 {
            n495 = local write "EXIT 2"(w921) -> ()
          }
          frame #6 {
            n496 = control-ref of="This Application"() -> (w936:refnum<vi>)
            n497 = property class="App"(reference=w936) -> ("App.Kind"=w935:T12)  [unwired: 1 in, 2 out]
            n498 = control-ref of="This VI"() -> (w929:refnum<vi>)
            n499 = Get Date/Time In Seconds() -> (seconds since 1Jan1904=w924:timestamp)
            n500 = case shown="\"Run Time System\"" w935 {
              frame "Development System", Default {
              }
              frame "Run Time System" {
                n501 = control-ref of="This VI"() -> (w942:refnum<vi>)
                n502 = invoke class="VI" method="FP.Close"(reference=w942) -> ()  [unwired: 2 in, 3 out]
                n503 = Quit LabVIEW() -> ()  [unwired: 1 in]
              }
            }
            n504 = property class="VI"(reference=w929) -> ("Path"=w928:path)  [unwired: 1 in, 2 out]
            n505 = Format Date/Time String(time format string (%c)="%d%m%y %I-%M %p ", seconds (now)=w924) -> (date/time string=w926:string)  [unwired: 1 in]
            n506 = Concatenate Strings(w926, "Log File.txt") -> (w930:string)
            n507 = Strip Path(path=w928) -> (stripped path=w931:path)  [unwired: 1 out]
            n508 = Build Path(base path=w931, name or relative path=w930) -> (appended path=w923:path)
            n509 = Open/Create/Replace File(file path (use dialog)=w923, operation (0:open)=T10."replace or create") -> (refnum out=w933:refnum<file>, cancelled=w934:bool, error out=w932:errorcluster)  [unwired: 4 in]
            n510 = case shown="False" w934 {
              tunnel: w933 -> [w941 _]
              tunnel: w932 -> [w939 _]
              frame False {
                n511 = local read "Log"() -> (w940:string)
                n512 = Write to Text File(file (use dialog)=w941, text=w940, error in=w939) -> (refnum out=w938:refnum<file>, error out=w937:errorcluster)  [unwired: 2 out]
                n513 = Close File(refnum=w938, error in=w937) -> ()  [unwired: 2 out]
              }
              frame True {
              }
            }
          }
          frame #7 {
          }
        }
      }
      event "Overlay MSI Image": Value Change {
        n514 = event-data() -> ()  [unwired: 1 in, 6 out]
        n515 = case shown="True" "Overlay MSI Image" {
          frame False {
          }
          frame True {
            n516 = vi-ref "MSI_Image_overlap.vi"() -> (w950:refnum<vi>)
            n517 = invoke class="VI" method="FP.Open"(reference=w950, "Activate"=TRUE ("Activate?"), "State"=T11."Standard") -> (reference out=w947:refnum<vi>)  [unwired: 2 in, 4 out]
            n518 = invoke class="VI" method="Run VI"(reference=w947, "Wait until done"=FALSE ("Wait Until Done"), "Auto Dispose Ref"=TRUE ("Auto Dispose Reference")) -> ()  [unwired: 2 in, 5 out]
          }
        }
      }
      event "Alignment \ndiode": Value Change {
        n519 = event-data() -> ()  [unwired: 1 in, 6 out]
        n520 = case shown="False" "Alignment \ndiode" {
          frame False {
            n521 = call "IR_Alignment_Diode.vi"("AD Action"=enum16{"AD Off", "AD On"}."AD Off") -> ()  [unwired: 14 in, 1 out]